vi "Dresden R2R Sputter 03.02.2018 IY24.vi"() -> ()   [LabVIEW 2009] (continued)
                                }
                                }
                                n18545 = local read "Semi"() -> (w25084:bool)
                                n18546 = Or(x=w25083, y=w25084) -> (x .or. y?=w25082:bool)
                                }
                                }
                                frame #1 {
                                }
                                }
                                }
                                frame #1 {
                                n18547 = local read "Semi"() -> (w25095:bool)
                                n18548 = case shown="False" w25095 {
                                frame #0 {
                                n18549 = Wait (ms)(milliseconds to wait=u32 1000) -> ()  [unwired: 1 out]
                                n18550 = local write "Ch2_Sd3"(TRUE ("Ch1_Sd1 2")) -> ()
                                }
                                frame #1 {
                                }
                                }
                                }
                                }
                                }
                                frame #1 {
                                }
                                }
                              }
                              frame #4 {
                                n18551 = local read "Yes 2"() -> (w25098:bool)
                                n18552 = case shown="False" w25098 {
                                frame #0 {
                                # "CLOSE PC-BV"
                                n18553 = local read "Semi"() -> (w25099:bool)
                                n18554 = case shown="False" w25099 {
                                frame #0 {
                                n18555 = stacked-sequence {
                                frame #0 {
                                n18556 = local read "Semi"() -> (w25100:bool)
                                n18557 = case shown="False" w25100 {
                                frame #0 {
                                n18558 = stacked-sequence {
                                frame #0 {
                                n18559 = local read "Semi"() -> (w25101:bool)
                                n18560 = case shown="False" w25101 {
                                frame #0 {
                                n18561 = local write "Pc_bv2_auto_close"(TRUE ("Tp1_auto_start")) -> ()
                                }
                                frame #1 {
                                }
                                }
                                }
                                frame #1 {
                                n18562 = local read "Semi"() -> (w25103:bool)
                                n18563 = case shown="False" w25103 {
                                frame #0 {
                                n18564 = Wait (ms)(milliseconds to wait=u32 1000) -> ()  [unwired: 1 out]
                                }
                                frame #1 {
                                }
                                }
                                }
                                frame #2 {
                                n18565 = local read "Semi"() -> (w25105:bool)
                                n18566 = case shown="False" w25105 {
                                frame #0 {
                                n18567 = while {
                                i -> [w25111]
                                stop <- w25107 stop-if-true
                                n18568 = local read "Pc_bv_closed_ch2"() -> (w25109:bool)
                                n18569 = Greater?(x=w25111, y=120) -> (0:w25110:bool)
                                n18570 = local read "Semi"() -> (w25108:bool)
                                n18571 = Compound Arithmetic op=OR(w25108, w25109, w25110) -> (w25107:bool)
                                n18572 = Wait (ms)(milliseconds to wait=u32 500) -> ()  [unwired: 1 out]
                                }
                                }
                                frame #1 {
                                }
                                }
                                }
                                frame #3 {
                                n18573 = local read "Semi"() -> (w25113:bool)
                                n18574 = case shown="False" w25113 {
                                frame #0 {
                                n18575 = local read "Pc_bv_closed_ch2"() -> (w25114:bool)
                                n18576 = case shown="False" w25114 {
                                frame #0 {
                                n18577 = local write "Pc_bv2_auto_close"(TRUE ("Pc_bv1_auto_open")) -> ()
                                }
                                frame #1 {
                                }
                                }
                                }
                                frame #1 {
                                }
                                }
                                }
                                frame #4 {
                                n18578 = local read "Semi"() -> (w25116:bool)
                                n18579 = case shown="False" w25116 {
                                frame #0 {
                                n18580 = local read "Pc_bv_closed_ch2"() -> (w25117:bool)
                                n18581 = case shown="False" w25117 {
                                frame #0 {
                                n18582 = Wait (ms)(milliseconds to wait=u32 1000) -> ()  [unwired: 1 out]
                                }
                                frame #1 {
                                }
                                }
                                }
                                frame #1 {
                                }
                                }
                                }
                                frame #5 {
                                n18583 = local read "Semi"() -> (w25119:bool)
                                n18584 = case shown="False" w25119 {
                                frame #0 {
                                n18585 = while {
                                i -> [w25125]
                                stop <- w25121 stop-if-true
                                n18586 = local read "Pc_bv_closed_ch2"() -> (w25123:bool)
                                n18587 = Greater?(x=w25125, y=120) -> (0:w25124:bool)
                                n18588 = local read "Semi"() -> (w25122:bool)
                                n18589 = Compound Arithmetic op=OR(w25122, w25123, w25124) -> (w25121:bool)
                                n18590 = Wait (ms)(milliseconds to wait=u32 500) -> ()  [unwired: 1 out]
                                }
                                }
                                frame #1 {
                                }
                                }
                                }
                                frame #6 {
                                n18591 = local read "Semi"() -> (w25127:bool)
                                n18592 = case shown="False" w25127 {
                                frame #0 {
                                n18593 = local read "Pc_bv_closed_ch2"() -> (w25128:bool)
                                n18594 = case shown="False" w25128 {
                                frame #0 {
                                n18595 = local write "Error Message"("Shut Down process  cancelled\nbecause  PC-BV not opened.\nPlease check PC-BV2 connections." ("Error Message")) -> ()
                                n18596 = local write "Semi"(TRUE ("Semi")) -> ()
                                }
                                frame #1 {
                                }
                                }
                                }
                                frame #1 {
                                }
                                }
                                }
                                }
                                }
                                frame #1 {
                                }
                                }
                                }
                                frame #1 {
                                n18597 = local read "Semi"() -> (w25131:bool)
                                n18598 = case shown="False" w25131 {
                                frame #0 {
                                n18599 = Wait (ms)(milliseconds to wait=u32 1000) -> ()  [unwired: 1 out]
                                n18600 = local write "Ch2_Sd4"(TRUE ("Ch1_Sd2")) -> ()
                                }
                                frame #1 {
                                }
                                }
                                }
                                }
                                }
                                frame #1 {
                                }
                                }
                                }
                                frame #1 {
                                # "OPEN PC-BV"
                                n18601 = local read "Semi"() -> (w25134:bool)
                                n18602 = case shown="False" w25134 {
                                frame #0 {
                                n18603 = stacked-sequence {
                                frame #0 {
                                n18604 = local read "Semi"() -> (w25135:bool)
                                n18605 = case shown="False" w25135 {
                                frame #0 {
                                n18606 = stacked-sequence {
                                frame #0 {
                                n18607 = local read "Semi"() -> (w25136:bool)
                                n18608 = case shown="False" w25136 {
                                frame #0 {
                                n18609 = local write "Pc_bv2_auto_open"(TRUE ("Tp1_auto_start")) -> ()
                                }
                                frame #1 {
                                }
                                }
                                }
                                frame #1 {
                                n18610 = local read "Semi"() -> (w25138:bool)
                                n18611 = case shown="False" w25138 {
                                frame #0 {
                                n18612 = Wait (ms)(milliseconds to wait=u32 1000) -> ()  [unwired: 1 out]
                                }
                                frame #1 {
                                }
                                }
                                }
                                frame #2 {
                                n18613 = local read "Semi"() -> (w25140:bool)
                                n18614 = case shown="False" w25140 {
                                frame #0 {
                                n18615 = while {
                                i -> [w25146]
                                stop <- w25142 stop-if-true
                                n18616 = local read "Pc_bv_opened_ch2"() -> (w25144:bool)
                                n18617 = Greater?(x=w25146, y=120) -> (0:w25145:bool)
                                n18618 = local read "Semi"() -> (w25143:bool)
                                n18619 = Compound Arithmetic op=OR(w25143, w25144, w25145) -> (w25142:bool)
                                n18620 = Wait (ms)(milliseconds to wait=u32 500) -> ()  [unwired: 1 out]
                                }
                                }
                                frame #1 {
                                }
                                }
                                }
                                frame #3 {
                                n18621 = local read "Semi"() -> (w25148:bool)
                                n18622 = case shown="False" w25148 {
                                frame #0 {
                                n18623 = local read "Pc_bv_opened_ch2"() -> (w25149:bool)
                                n18624 = case shown="False" w25149 {
                                frame #0 {
                                n18625 = local write "Pc_bv2_auto_open"(TRUE ("Pc_bv1_auto_open")) -> ()
                                }
                                frame #1 {
                                }
                                }
                                }
                                frame #1 {
                                }
                                }
                                }
                                frame #4 {
                                n18626 = local read "Semi"() -> (w25151:bool)
                                n18627 = case shown="False" w25151 {
                                frame #0 {
                                n18628 = local read "Pc_bv_opened_ch2"() -> (w25152:bool)
                                n18629 = case shown="False" w25152 {
                                frame #0 {
                                n18630 = Wait (ms)(milliseconds to wait=u32 1000) -> ()  [unwired: 1 out]
                                }
                                frame #1 {
                                }
                                }
                                }
                                frame #1 {
                                }
                                }
                                }
                                frame #5 {
                                n18631 = local read "Semi"() -> (w25154:bool)
                                n18632 = case shown="False" w25154 {
                                frame #0 {
                                n18633 = while {
                                i -> [w25160]
                                stop <- w25156 stop-if-true
                                n18634 = local read "Pc_bv_opened_ch2"() -> (w25158:bool)
                                n18635 = Greater?(x=w25160, y=120) -> (0:w25159:bool)
                                n18636 = local read "Semi"() -> (w25157:bool)
                                n18637 = Compound Arithmetic op=OR(w25157, w25158, w25159) -> (w25156:bool)
                                n18638 = Wait (ms)(milliseconds to wait=u32 500) -> ()  [unwired: 1 out]
                                }
                                }
                                frame #1 {
                                }
                                }
                                }
                                frame #6 {
                                n18639 = local read "Semi"() -> (w25162:bool)
                                n18640 = case shown="False" w25162 {
                                frame #0 {
                                n18641 = local read "Pc_bv_opened_ch2"() -> (w25163:bool)
                                n18642 = case shown="False" w25163 {
                                frame #0 {
                                n18643 = local write "Error Message"("Shut Down process  cancelled\nbecause  PC-BV not opened.\nPlease check PC-BV2 connections." ("Error Message")) -> ()
                                n18644 = Wait (ms)(milliseconds to wait=u32 1000) -> ()  [unwired: 1 out]
                                }
                                frame #1 {
                                }
                                }
                                }
                                frame #1 {
                                }
                                }
                                }
                                }
                                }
                                frame #1 {
                                }
                                }
                                }
                                frame #1 {
                                n18645 = local read "Semi"() -> (w25166:bool)
                                n18646 = case shown="False" w25166 {
                                frame #0 {
                                n18647 = Wait (ms)(milliseconds to wait=u32 1000) -> ()  [unwired: 1 out]
                                n18648 = local write "Ch2_Sd5"(TRUE ("Ch1_Sd2")) -> ()
                                }
                                frame #1 {
                                }
                                }
                                }
                                }
                                }
                                frame #1 {
                                }
                                }
                                }
                                }
                              }
                              frame #5 {
                                # "CLOSE TP-BV"
                                n18649 = local read "Semi"() -> (w25169:bool)
                                n18650 = case shown="False" w25169 {
                                frame #0 {
                                n18651 = stacked-sequence {
                                frame #0 {
                                n18652 = local read "Semi"() -> (w25170:bool)
                                n18653 = case shown="False" w25170 {
                                frame #0 {
                                n18654 = while {
                                i -> [w25176]
                                stop <- w25171 stop-if-true
                                n18655 = Greater?(x=w25176, y=25) -> (0:w25175:bool)
                                n18656 = case shown="True" w25175 {
                                frame #0 {
                                }
                                frame #1 {
                                n18657 = local write "Error Message"("Shut Down Process  cancelled\nbecause  TP-BV not closed.\nPlease check TP-BV2 connections." ("Error Message")) -> ()
                                n18658 = local write "Semi"(TRUE ("Semi")) -> ()
                                }
                                }
                                n18659 = local read "Ch2_Tp_bv_di"() -> (w25174:bool)
                                n18660 = case shown="True" w25174 {
                                tunnel: [TRUE FALSE] -> w25172
                                frame #0 {
                                }
                                frame #1 {
                                n18661 = Wait Until Next ms Multiple(millisecond multiple=u32 200) -> ()  [unwired: 1 out]
                                n18662 = local write "Ch2_Tp_bv_do"(FALSE ("Ch1_Ch_cc_on_off_di")) -> ()
                                }
                                }
                                n18663 = local read "Semi"() -> (w25173:bool)
                                n18664 = Or(x=w25172, y=w25173) -> (x .or. y?=w25171:bool)
                                }
                                }
                                frame #1 {
                                }
                                }
                                }
                                frame #1 {
                                n18665 = local read "Semi"() -> (w25184:bool)
                                n18666 = case shown="False" w25184 {
                                frame #0 {
                                n18667 = local write "Ch2_Sd6"(TRUE ("Ch1_Sd5")) -> ()
                                n18668 = Wait (ms)(milliseconds to wait=u32 1000) -> ()  [unwired: 1 out]
                                }
                                frame #1 {
                                }
                                }
                                }
                                }
                                }
                                frame #1 {
                                }
                                }
                              }
                              frame #6 {
                                # "STOP MP"
                                n18669 = local read "Semi"() -> (w25187:bool)
                                n18670 = case shown="False" w25187 {
                                frame #0 {
                                n18671 = stacked-sequence {
                                frame #0 {
                                n18672 = local read "Semi"() -> (w25188:bool)
                                n18673 = case shown="False" w25188 {
                                frame #0 {
                                n18674 = while {
                                i -> [w25194]
                                stop <- w25189 stop-if-true
                                n18675 = Greater?(x=w25194, y=25) -> (0:w25193:bool)
                                n18676 = case shown="True" w25193 {
                                frame #0 {
                                }
                                frame #1 {
                                n18677 = local write "Error Message"("Shut Down Process  cancelled\nbecause  MP not closed.\nPlease check MP2 connections." ("Error Message")) -> ()
                                n18678 = local write "Semi"(TRUE ("Semi")) -> ()
                                }
                                }
                                n18679 = local read "Ch2_Mp_di"() -> (w25192:bool)
                                n18680 = case shown="True" w25192 {
                                tunnel: [TRUE FALSE] -> w25190
                                frame #0 {
                                }
                                frame #1 {
                                n18681 = Wait Until Next ms Multiple(millisecond multiple=u32 200) -> ()  [unwired: 1 out]
                                n18682 = local write "Ch2_Mp_do"(FALSE ("Ch1_Ch_cc_on_off_di")) -> ()
                                }
                                }
                                n18683 = local read "Semi"() -> (w25191:bool)
                                n18684 = Or(x=w25190, y=w25191) -> (x .or. y?=w25189:bool)
                                }
                                }
                                frame #1 {
                                }
                                }
                                }
                                frame #1 {
                                n18685 = local read "Semi"() -> (w25202:bool)
                                n18686 = case shown="False" w25202 {
                                frame #0 {
                                n18687 = local write "Ch2_Sd7"(TRUE ("Ch1_Sd6")) -> ()
                                n18688 = Wait (ms)(milliseconds to wait=u32 1000) -> ()  [unwired: 1 out]
                                }
                                frame #1 {
                                }
                                }
                                }
                                }
                                }
                                frame #1 {
                                }
                                }
                              }
                              frame #7 {
                                # "PL-VBV OPEN  & CHECK"
                                n18689 = local read "Semi"() -> (w25205:bool)
                                n18690 = case shown="False" w25205 {
                                frame #0 {
                                n18691 = stacked-sequence {
                                frame #0 {
                                n18692 = local read "Semi"() -> (w25206:bool)
                                n18693 = case shown="False" w25206 {
                                frame #0 {
                                n18694 = local write "Ch2_Pl_atm_do"(FALSE ("Ch1_Pl_atm_do")) -> ()
                                n18695 = Wait Until Next ms Multiple(millisecond multiple=u32 2000) -> ()  [unwired: 1 out]
                                }
                                frame #1 {
                                }
                                }
                                }
                                frame #1 {
                                n18696 = local read "Semi"() -> (w25209:bool)
                                n18697 = case shown="False" w25209 {
                                frame #0 {
                                n18698 = while {
                                i -> [w25215]
                                stop <- w25211 stop-if-true
                                n18699 = Greater?(x=w25215, y=50) -> (0:w25214:bool)
                                n18700 = case shown="True" w25214 {
                                frame #0 {
                                }
                                frame #1 {
                                n18701 = local write "Error Message"("Shut Down Process  cancelled\nbecause  PL-VBV not opened.\nPlease check  PL-VBV2 connections." ("Error Message")) -> ()
                                n18702 = local write "Semi"(TRUE ("Semi")) -> ()
                                }
                                }
                                n18703 = local read "Ch2_Pl_atm_di"() -> (w25210:bool)
                                n18704 = case shown="False" w25210 {
                                tunnel: [w25217 TRUE] -> w25212
                                frame #0 {
                                n18705 = local read "Ch2_Pl_vbv_di"() -> (w25218:bool)
                                n18706 = case shown="False" w25218 {
                                tunnel: [FALSE TRUE] -> w25217
                                frame #0 {
                                n18707 = Wait Until Next ms Multiple(millisecond multiple=u32 500) -> ()  [unwired: 1 out]
                                n18708 = local write "Ch2_Pl_vbv_do"(TRUE ("Ch1_Ch_cc_on_off_di")) -> ()
                                }
                                frame #1 {
                                }
                                }
                                }
                                frame #1 {
                                n18709 = Wait Until Next ms Multiple(millisecond multiple=u32 500) -> ()  [unwired: 1 out]
                                }
                                }
                                n18710 = local read "Semi"() -> (w25213:bool)
                                n18711 = Or(x=w25212, y=w25213) -> (x .or. y?=w25211:bool)
                                }
                                }
                                frame #1 {
                                }
                                }
                                }
                                frame #2 {
                                n18712 = local read "Semi"() -> (w25227:bool)
                                n18713 = case shown="False" w25227 {
                                frame #0 {
                                n18714 = local write "Ch2_Sd8"(FALSE ("Ch1_Sd8")) -> ()
                                n18715 = Wait (ms)(milliseconds to wait=u32 1000) -> ()  [unwired: 1 out]
                                }
                                frame #1 {
                                }
                                }
                                }
                                }
                                }
                                frame #1 {
                                }
                                }
                              }
                              frame #8 {
                                # "PL-VBV CLOSE  & CHECK"
                                n18716 = local read "Semi"() -> (w25230:bool)
                                n18717 = case shown="False" w25230 {
                                frame #0 {
                                n18718 = stacked-sequence {
                                frame #0 {
                                n18719 = local read "Semi"() -> (w25231:bool)
                                n18720 = case shown="False" w25231 {
                                frame #0 {
                                n18721 = while {
                                i -> [w25237]
                                stop <- w25233 stop-if-true
                                n18722 = Greater?(x=w25237, y=50) -> (0:w25236:bool)
                                n18723 = case shown="True" w25236 {
                                frame #0 {
                                }
                                frame #1 {
                                n18724 = local write "Error Message"("Shut Down Process  cancelled\nbecause  PL-VBV not closed.\nPlease check PL-VBV2 connections." ("Error Message")) -> ()
                                n18725 = local write "Semi"(TRUE ("Semi")) -> ()
                                }
                                }
                                n18726 = local read "Ch2_Pl_atm_di"() -> (w25232:bool)
                                n18727 = case shown="True" w25232 {
                                tunnel: [FALSE w25241] -> w25234
                                frame #0 {
                                n18728 = Wait Until Next ms Multiple(millisecond multiple=u32 500) -> ()  [unwired: 1 out]
                                }
                                frame #1 {
                                n18729 = local read "Ch2_Pl_vbv_di"() -> (w25242:bool)
                                n18730 = case shown="True" w25242 {
                                tunnel: [TRUE FALSE] -> w25241
                                frame #0 {
                                }
                                frame #1 {
                                n18731 = Wait Until Next ms Multiple(millisecond multiple=u32 500) -> ()  [unwired: 1 out]
                                n18732 = local write "Ch2_Pl_vbv_do"(FALSE ("Ch1_Ch_cc_on_off_di")) -> ()
                                }
                                }
                                }
                                }
                                n18733 = local read "Semi"() -> (w25235:bool)
                                n18734 = Or(x=w25234, y=w25235) -> (x .or. y?=w25233:bool)
                                }
                                }
                                frame #1 {
                                }
                                }
                                }
                                frame #1 {
                                n18735 = local read "Semi"() -> (w25249:bool)
                                n18736 = case shown="False" w25249 {
                                frame #0 {
                                n18737 = local write "Ch2_Sd9"(TRUE ("Ch1_Sd11")) -> ()
                                n18738 = Wait (ms)(milliseconds to wait=u32 1000) -> ()  [unwired: 1 out]
                                }
                                frame #1 {
                                }
                                }
                                }
                                }
                                }
                                frame #1 {
                                }
                                }
                              }
                              frame #9 {
                                # "WAIT DECELARATING TP"
                                n18739 = local read "Semi"() -> (w25252:bool)
                                n18740 = case shown="False" w25252 {
                                frame #0 {
                                n18741 = stacked-sequence {
                                frame #0 {
                                n18742 = local read "Semi"() -> (w25253:bool)
                                n18743 = case shown="False" w25253 {
                                frame #0 {
                                n18744 = while {
                                i -> [w25259]
                                stop <- w25255 stop-if-true
                                n18745 = Greater?(x=w25259, y=1500) -> (0:w25258:bool)
                                n18746 = case shown="True" w25258 {
                                frame #0 {
                                }
                                frame #1 {
                                n18747 = local write "Error Message"("Shut Down Process  cancelled\nbecause TP not decelarating.\nPlease check TP2 connections." ("Error Message")) -> ()
                                n18748 = local write "Semi"(TRUE ("Semi")) -> ()
                                }
                                }
                                n18749 = local read "Yes 2"() -> (w25254:bool)
                                n18750 = case shown="True" w25254 {
                                tunnel: [TRUE w25265] -> w25256
                                frame #0 {
                                }
                                frame #1 {
                                n18751 = local read "Tp2_speed_gui"() -> (w25263:i32)
                                n18752 = Less?(x=w25263, y="Tp2_safety_speed") -> (x < y?=w25262:bool)
                                n18753 = case shown="False" w25262 {
                                tunnel: [FALSE TRUE] -> w25265
                                frame #0 {
                                n18754 = Wait Until Next ms Multiple(millisecond multiple=u32 500) -> ()  [unwired: 1 out]
                                }
                                frame #1 {
                                }
                                }
                                }
                                }
                                n18755 = local read "Semi"() -> (w25257:bool)
                                n18756 = Or(x=w25256, y=w25257) -> (x .or. y?=w25255:bool)
                                }
                                }
                                frame #1 {
                                }
                                }
                                }
                                frame #1 {
                                n18757 = local read "Semi"() -> (w25271:bool)
                                n18758 = case shown="False" w25271 {
                                frame #0 {
                                n18759 = Wait (ms)(milliseconds to wait=u32 1000) -> ()  [unwired: 1 out]
                                n18760 = local write "Ch2_Sd10"(TRUE ("Ch1_Sd3")) -> ()
                                }
                                frame #1 {
                                }
                                }
                                }
                                }
                                }
                                frame #1 {
                                }
                                }
                              }
                              frame #10 {
                                # "CH-VBV OPEN  & CHECK"
                                n18761 = local read "Yes 2"() -> (w25274:bool)
                                n18762 = case shown="True" w25274 {
                                frame #0 {
                                }
                                frame #1 {
                                n18763 = local read "Semi"() -> (w25275:bool)
                                n18764 = case shown="False" w25275 {
                                frame #0 {
                                n18765 = stacked-sequence {
                                frame #0 {
                                n18766 = local read "Semi"() -> (w25276:bool)
                                n18767 = case shown="False" w25276 {
                                frame #0 {
                                n18768 = local write "Ch2_Ch_atm_do"(FALSE ("Ch1_Pl_atm_do")) -> ()
                                n18769 = Wait Until Next ms Multiple(millisecond multiple=u32 2000) -> ()  [unwired: 1 out]
                                }
                                frame #1 {
                                }
                                }
                                }
                                frame #1 {
                                n18770 = local read "Semi"() -> (w25279:bool)
                                n18771 = case shown="False" w25279 {
                                frame #0 {
                                n18772 = while {
                                i -> [w25285]
                                stop <- w25281 stop-if-true
                                n18773 = Greater?(x=w25285, y=50) -> (0:w25284:bool)
                                n18774 = case shown="True" w25284 {
                                frame #0 {
                                }
                                frame #1 {
                                n18775 = local write "Error Message"("Shut Down Process  cancelled\nbecause  CH-VBV not opened.\nPlease check  CH-VBV2 connections." ("Error Message")) -> ()
                                n18776 = local write "Semi"(TRUE ("Semi")) -> ()
                                }
                                }
                                n18777 = local read "Ch2_Ch_atm_di"() -> (w25280:bool)
                                n18778 = case shown="False" w25280 {
                                tunnel: [w25287 TRUE] -> w25282
                                frame #0 {
                                n18779 = local read "Ch2_Ch_vbv_di"() -> (w25288:bool)
                                n18780 = case shown="False" w25288 {
                                tunnel: [FALSE TRUE] -> w25287
                                frame #0 {
                                n18781 = Wait Until Next ms Multiple(millisecond multiple=u32 200) -> ()  [unwired: 1 out]
                                n18782 = local write "Ch2_Ch_vbv_do"(TRUE ("Ch1_Ch_cc_on_off_di")) -> ()
                                }
                                frame #1 {
                                }
                                }
                                }
                                frame #1 {
                                }
                                }
                                n18783 = local read "Semi"() -> (w25283:bool)
                                n18784 = Or(x=w25282, y=w25283) -> (x .or. y?=w25281:bool)
                                }
                                }
                                frame #1 {
                                }
                                }
                                }
                                frame #2 {
                                n18785 = local read "Semi"() -> (w25296:bool)
                                n18786 = case shown="False" w25296 {
                                frame #0 {
                                n18787 = local write "Ch2_Sd11"(TRUE ("Ch1_Sd9")) -> ()
                                n18788 = Wait (ms)(milliseconds to wait=u32 1000) -> ()  [unwired: 1 out]
                                }
                                frame #1 {
                                }
                                }
                                }
                                }
                                }
                                frame #1 {
                                }
                                }
                                }
                                }
                              }
                              frame #11 {
                                # "CH-VBV CLOSE &  CHECK"
                                n18789 = local read "Yes 2"() -> (w25299:bool)
                                n18790 = case shown="True" w25299 {
                                frame #0 {
                                }
                                frame #1 {
                                n18791 = local read "Semi"() -> (w25300:bool)
                                n18792 = case shown="False" w25300 {
                                frame #0 {
                                n18793 = stacked-sequence {
                                frame #0 {
                                n18794 = local read "Semi"() -> (w25301:bool)
                                n18795 = case shown="False" w25301 {
                                frame #0 {
                                n18796 = while {
                                i -> [w25309]
                                stop <- w25305 stop-if-true
                                n18797 = Greater?(x=w25309, y=50) -> (0:w25308:bool)
                                n18798 = case shown="True" w25308 {
                                frame #0 {
                                }
                                frame #1 {
                                n18799 = local write "Error Message"("Shut Down Process  cancelled\nbecause  CH-VBV  not closed.\nPlease check CH-VBV2 connections." ("Error Message")) -> ()
                                n18800 = local write "Semi"(TRUE ("Semi")) -> ()
                                }
                                }
                                n18801 = local read "Tp2_speed_gui"() -> (w25303:i32)
                                n18802 = Greater Or Equal?(x=w25303, y=u64 100) -> (x >= y?=w25302:bool)
                                n18803 = case shown="True" w25302 {
                                tunnel: [TRUE w25312] -> w25306
                                frame #0 {
                                }
                                frame #1 {
                                n18804 = local read "Ch2_Ch_vbv_di"() -> (w25313:bool)
                                n18805 = case shown="True" w25313 {
                                tunnel: [TRUE FALSE] -> w25312
                                frame #0 {
                                }
                                frame #1 {
                                n18806 = Wait Until Next ms Multiple(millisecond multiple=u32 500) -> ()  [unwired: 1 out]
                                n18807 = local write "Ch2_Ch_vbv_do"(FALSE ("Ch1_Ch_cc_on_off_di")) -> ()
                                }
                                }
                                }
                                }
                                n18808 = local read "Semi"() -> (w25307:bool)
                                n18809 = Or(x=w25306, y=w25307) -> (x .or. y?=w25305:bool)
                                }
                                }
                                frame #1 {
                                }
                                }
                                }
                                frame #1 {
                                n18810 = local read "Semi"() -> (w25320:bool)
                                n18811 = case shown="False" w25320 {
                                frame #0 {
                                n18812 = local write "Ch2_Sd12"(TRUE ("Ch1_Sd13")) -> ()
                                n18813 = Wait (ms)(milliseconds to wait=u32 1000) -> ()  [unwired: 1 out]
                                }
                                frame #1 {
                                }
                                }
                                }
                                frame #2 {
                                n18814 = local read "Semi"() -> (w25323:bool)
                                n18815 = case shown="False" w25323 {
                                frame #0 {
                                n18816 = Wait (ms)(milliseconds to wait=u32 3000) -> ()  [unwired: 1 out]
                                }
                                frame #1 {
                                }
                                }
                                }
                                }
                                }
                                frame #1 {
                                }
                                }
                                }
                                }
                              }
                              frame #12 {
                                # "CH-VBV OPEN &  CHECK"
                                n18817 = local read "Yes 2"() -> (w25325:bool)
                                n18818 = case shown="True" w25325 {
                                frame #0 {
                                }
                                frame #1 {
                                n18819 = local read "Semi"() -> (w25326:bool)
                                n18820 = case shown="False" w25326 {
                                frame #0 {
                                n18821 = stacked-sequence {
                                frame #0 {
                                n18822 = local read "Semi"() -> (w25327:bool)
                                n18823 = case shown="False" w25327 {
                                frame #0 {
                                n18824 = while {
                                i -> [w25333]
                                stop <- w25329 stop-if-true
                                n18825 = Greater?(x=w25333, y=200) -> (0:w25332:bool)
                                n18826 = case shown="True" w25332 {
                                frame #0 {
                                }
                                frame #1 {